vi "UHR-Fleezers Control (host) - 12.7e.vi"() -> ()   [LabVIEW 2012] (continued)
        n2981 = xnode "Read/Write Control"("FPGA VI Reference In"=w4045, "error in"=w4044) -> ("FPGA VI Reference Out"=w4043:T20, "error out"=w4042:errorcluster, "APD 3 Gate Late Counter"=→"APD 3 Gate Late Counter":u8, "APD 3 Gate Relative Phase"=→"APD 3 Gate Relative Phase":i16)
      }
    }
    n2982 = Not Equal?(x=w3728, y="Calibration") -> (x != y?=w3687:bool)
    n2983 = case shown="True" w3687 {
      tunnel: w3726 -> [_ w4076]
      tunnel: w3725 -> [_ w4075]
      tunnel: w3724 -> [_ w4074]
      tunnel: w3721 -> [_ w4073]
      tunnel: w3661 -> [_ w4072]
      frame False {
      }
      frame True {
        n2984 = property on="Force" class="WFChart (strict)"("YScale.NameLbl.Text"=w4076) -> ()  [unwired: 2 in, 2 out]
        n2985 = property on="T2 X" class="DigNum (strict)"("Caption.Text"=w4074) -> ()  [unwired: 2 in, 2 out]
        n2986 = property on="T1 X" class="DigNum (strict)"("Caption.Text"=w4075) -> ()  [unwired: 2 in, 2 out]
        n2987 = property on="Mean" class="DigNum (strict)"("Caption.Text"=w4073) -> ()  [unwired: 2 in, 2 out]
        n2988 = property on="Difference" class="DigNum (strict)"("Caption.Text"=w4072) -> ()  [unwired: 2 in, 2 out]
      }
    }
    n2989 = Unbundle By Name(w3709) -> ("Y"=w3712:dbl[])
    n2990 = Unbundle By Name(w3706) -> ("Y"=w3715:dbl[])
    n2991 = Subtract(x=w3712, y=w3710) -> (x-y=w3713:dbl[])
    n2992 = Subtract(x=w3715, y=w3708) -> (x-y=w3714:dbl[])
    n2993 = Multiply(x=w3714, y="T2 alpha_x (nm/V)") -> (x*y=w3510:dbl[])
    n2994 = Multiply(x="T1 alpha_x (nm/V)", y=w3713) -> (x*y=w3511:dbl[])
    n2995 = Not(x="Trap Trig. Fl.") -> (.not. x?=w3547:bool)
    n2996 = Multiply(x=w3736, y=-1.0) -> (x*y=w3717:waveform(dbl))
    n2997 = Subtract(x=w3511, y=w3510) -> (x-y=w3705:dbl[])
    n2998 = Unbundle By Name(w3736) -> ("Y"=w3677:dbl[])
    n2999 = Unbundle By Name(w3737) -> ("Y"=w3512:dbl[])
    n3000 = Negate(x=w3705) -> (-x=w3508:dbl[])
    n3001 = Build Array(w3737, w3717) -> (→"Force":waveform(dbl)[])
    n3002 = Subtract(x=w3508, y="Offset (nm)") -> (x-y=w3675:dbl[])
    n3003 = call-poly <vilib>:"Mean.vi"("X"=w3677) -> ("mean"=w3514:dbl)  [unwired: 1 out]
    "T2 X" <- w3514
    n3004 = Negate(x=w3677) -> (-x=w3678:dbl[])
    n3005 = call-poly <vilib>:"Mean.vi"("X"=w3512) -> ("mean"=w3515:dbl)  [unwired: 1 out]
    "T1 X" <- w3515
    n3006 = Negate(x=w3514) -> (-x=w3513:dbl)
    n3007 = Bundle By Name(cluster=w3709, "Y"=w3675) -> (w3653:waveform(dbl))
    "Bead Separation" <- w3653
    n3008 = Add(x=w3512, y=w3678) -> (x+y=w3679:dbl[])
    n3009 = Add(x=w3515, y=w3513) -> (x+y=w3723:dbl)
    n3010 = Subtract(x=w3515, y=w3513) -> (x-y=→"Difference":dbl)
    n3011 = Divide(x=w3679, y=2.0) -> (x/y=→"Vec Mean of T1 T2":dbl[])
    n3012 = Divide(x=w3723, y=2.0) -> (x/y=w3681:dbl)
    "Mean" <- w3681
    n3013 = feedback-in #25("Trap Trig. Fl.") -> ()
    n3014 = feedback #25("Trap Trig. Fl.") -> (w3545:bool)
    n3015 = And(x=w3547, y=w3545) -> (x .and. y?=w3546:bool)
    n3016 = case "If have just turned off triggering" shown="True" w3546 {
      tunnel: w3528 -> [_ w3873]
      tunnel: w3527 -> [_ w3872]
      frame False {
      }
      frame True {
        w3871 = FALSE ("FPGA Trap Trig")
        n3017 = xnode "Read/Write Control"("FPGA VI Reference In"=w3873, "error in"=w3872, "FPGA Trap Trig"=w3871) -> ("FPGA VI Reference Out"=w3870:T20, "error out"=w3869:errorcluster)
        n3018 = xnode "Read/Write Control"("FPGA VI Reference In"=w3870, "error in"=w3869, "TTrig?"=w3871) -> ()  [unwired: 2 out]
        n3019 = local write "Initializing"(FALSE ("Initializing")) -> ()
        n3020 = local write "Triggered"(FALSE ("Triggered")) -> ()
        n3021 = local write "Waiting"(FALSE ("Waiting")) -> ()
      }
    }
    n3022 = Not(x=w3545) -> (.not. x?=w3558:bool)
    n3023 = And(x="Trap Trig. Fl.", y=w3558) -> (x .and. y?=w3555:bool)
    n3024 = local read "Tether"() -> (w3682:bool)
    n3025 = Or(x=w3555, y="Reinitialize") -> (x .or. y?=w3541:bool)
    n3026 = feedback #26(w3551) -> (w3556:string)
    n3027 = Select(t=w3551, s=w3555, f=w3556) -> (s? t:f=w3550:string)
    n3028 = Select(t=w3551, s="Reinitialize", f=w3550) -> (s? t:f=w3549:string)
    n3029 = feedback #27(0) -> (w3553:i32)
    n3030 = feedback #28(w3675) -> (w3674:dbl[])
    n3031 = Build Array (concatenate)(w3675, w3674) -> (w3509:dbl[])
    n3032 = case "For determining if there is a tether still" shown="True" w3682 {
      tunnel: w3681 -> [_ w3997]
      frame False {
      }
      frame True {
        n3033 = Greater?(x="Lost Tether Alarm Threshold (pN)", y=w3997) -> (0:w3995:bool)
        n3034 = case shown="True" w3995 {
          frame False {
          }
          frame True {
            w3998 = FALSE ("Value (Signaling)")
            n3035 = flat-sequence {
              frame #0 {
                # "stop only if saving"
                n3036 = local read "Saving..."() -> (w4010:bool)
                n3037 = And(x=w4010, y="TA Cancel Save?") -> (x .and. y?=w4009:bool)
                n3038 = local write "Stop Saving"(w4009) -> ()
              }
              frame #1 {
                n3039 = case shown="True" "TA Green Off?" {
                  frame False {
                  }
                  frame True {
                    w4013 = FALSE ("Fl. Triggered...")
                    n3040 = local write "Fl. Triggered..."(w4013) -> ()
                    n3041 = property on="Green Laser ON" class="Bool (strict)"("Val(Sgnl)"=w4013) -> ()  [unwired: 2 in, 2 out]
                  }
                }
              }
            }
            n3042 = local read "Time tether formed"() -> (w4004:timestamp)
            n3043 = Get Date/Time In Seconds() -> (seconds since 1Jan1904=w4005:timestamp)
            n3044 = Subtract(x=w4005, y=w4004) -> (x-y=w4003:dbl)
            n3045 = Number To Decimal String(number=w4003) -> (decimal integer string=w4000:string)  [unwired: 1 out]
            n3046 = local read "Messages"() -> (w4007:string)
            n3047 = call <vilib>:"Beep.vi"() -> ()  [unwired: 3 in, 9 out]
            n3048 = Concatenate Strings("Lost tether (" ("Message to add"), w4000, " s)." ("string")) -> (w4002:string)
            n3049 = local write "Tether"(FALSE ("Tether")) -> ()
            n3050 = call "Update messages.vi"("Message to add"=w4002, "Old message string"=w4007) -> ("New message string"=w4006:string)
            n3051 = local write "Messages"(w4006) -> ()
            n3052 = property on="Fl. Triggered..." class="Bool (strict)"("Val(Sgnl)"=w3998) -> ()  [unwired: 2 in, 2 out]
            n3053 = local write "Dip for Protein"(w3998) -> ()
            n3054 = property on="Trap Pos. FB ON" class="Bool (strict)"("Val(Sgnl)"=w3998) -> ()  [unwired: 2 in, 2 out]
            n3055 = property on="Trap Trig. Fl." class="Bool (strict)"("Val(Sgnl)"=w3998) -> ()  [unwired: 2 in, 2 out]
          }
        }
      }
    }
    n3056 = case "For triggering actions based on the trap position (e.g., turning the excitation laser on if trap under feedback moves so far)" shown="True" "Trap Trig. Fl." {
      tunnel: w3536 -> [_ w3886]
      tunnel: w3549 -> [_ w3885]
      tunnel: ["" ("t") w3884] -> w3557
      tunnel: w3541 -> [_ w3883]
      tunnel: [0 ("t") w3882] -> w3554
      tunnel: w3553 -> [_ w3881]
      tunnel: w3528 -> [_ w3880]
      tunnel: w3527 -> [_ w3879]
      frame False {
      }
      frame True {
        n3057 = case shown="\"Wait for trigger\"" w3885 {
          tunnel: w3886 -> [w3903 _ _ w3951]
          tunnel: [w3900 w3932 "" ("t") w3954] -> w3884
          tunnel: w3883 -> [_ _ _ w3942]
          tunnel: [w3899 w3929 0 ("t") w3943] -> w3882
          tunnel: w3881 -> [_ w3931 _ w3949]
          tunnel: w3880 -> [w3888 w3926 _ w3945]
          tunnel: w3879 -> [w3887 w3925 _ w3944]
          frame "Wait for trigger" {
            n3058 = local read "Trap Trig. (FPGA)"() -> (w3891:bool)
            n3059 = Subtract(x=w3903, y="Mean T1 Position\nto compare (nm)") -> (x-y=w3896:dbl[])
            n3060 = call <vilib>:"Std Deviation and Variance.vi"("X"=w3896) -> ("mean"=→"mean":dbl, "standard deviation"=→"standard\ndeviation":dbl)  [unwired: 1 in, 1 out]
            n3061 = Array Max & Min(array=w3896) -> (max value=→"max value":dbl, min value=→"min value":dbl)  [unwired: 2 out]
            n3062 = Greater?(x=w3896, y="Threshold (nm)") -> (0:w3906:bool[])
            n3063 = case shown="True" w3891 {
              tunnel: w3888 -> [_ w3912]
              tunnel: w3887 -> [_ w3911]
              tunnel: [FALSE ("TTrig?") w3910] -> w3894
              frame False {
              }
              frame True {
                n3064 = xnode "Read/Write Control"("FPGA VI Reference In"=w3912, "error in"=w3911) -> ("TTrig?"=w3910:bool)  [unwired: 2 out]
              }
            }
            n3065 = Or Array Elements(Boolean array=w3906) -> (logical OR=w3893:bool)
            n3066 = Select(t=w3894, s=w3891, f=w3893) -> (s? t:f=w3892:bool)
            n3067 = Not(x=w3891) -> (.not. x?=w3890:bool)
            n3068 = And(x=w3892, y=w3890) -> (x .and. y?=w3889:bool)
            n3069 = Select(t="Triggered", s=w3892, f="Wait for trigger") -> (s? t:f=w3900:string)
            n3070 = case shown="True" w3892 {
              tunnel: [0 0] -> w3899
              tunnel: w3888 -> [_ w3917]
              tunnel: w3887 -> [_ w3916]
              frame False {
                "Waiting" <- TRUE ("Waiting")
              }
              frame True {
                n3071 = xnode "Read/Write Control"("FPGA VI Reference In"=w3917, "error in"=w3916, "TTrig?"=FALSE) -> ()  [unwired: 2 out]
                n3072 = local read "Messages"() -> (w3920:string)
                n3073 = call <vilib>:"Beep.vi"() -> ()  [unwired: 12 in]
                n3074 = call "Update messages.vi"("Message to add"="Unwinding trigger.", "Old message string"=w3920) -> ("New message string"=w3921:string)
                n3075 = local write "Messages"(w3921) -> ()
                n3076 = local write "Waiting"(FALSE ("Waiting")) -> ()
                "Triggered" <- TRUE ("Triggered")
              }
            }
            n3077 = case "Only need to turn on laser if host triggered" shown="True" w3889 {
              frame False {
              }
              frame True {
                n3078 = property on="Green Laser ON" class="Bool (strict)"("Val(Sgnl)"=TRUE ("Value (Signaling)")) -> ()  [unwired: 2 in, 2 out]
              }
            }
          }
          frame "Triggered" {
            n3079 = local read "Trap Trig. (FPGA)"() -> (w3928:bool)
            n3080 = Increment(x=w3931) -> (x+1=w3929:i32)
            n3081 = Greater Or Equal?(x=w3929, y="Fl. ON time (n)") -> (x >= y?=w3927:bool)
            n3082 = Select(t="Wait for trigger", s=w3927, f="Triggered" ("t")) -> (s? t:f=w3932:string)
            n3083 = And(x=w3927, y=w3928) -> (x .and. y?=w3924:bool)
            n3084 = case shown="True" w3924 {
              tunnel: w3926 -> [_ w3936]
              tunnel: w3925 -> [_ w3935]
              frame False {
              }
              frame True {
                n3085 = xnode "Read/Write Control"("FPGA VI Reference In"=w3936, "error in"=w3935, "FPGA Trap Trig"=TRUE) -> ()  [unwired: 2 out]
              }
            }
            n3086 = case shown="True" w3927 {
              frame False {
              }
              frame True {
                w3938 = FALSE ("Value (Signaling)")
                n3087 = local write "Triggered"(w3938) -> ()
                n3088 = local write "Waiting"(TRUE ("Waiting")) -> ()
                n3089 = property on="Green Laser ON" class="Bool (strict)"("Val(Sgnl)"=w3938) -> ()  [unwired: 2 in, 2 out]
              }
            }
          }
          frame "Do nothing" {
          }
          frame "Initialize", Default {
            n3090 = Increment(x=w3949) -> (x+1=w3953:i32)
            n3091 = Select(t=1, s=w3942, f=w3953) -> (s? t:f=w3943:i32)
            n3092 = feedback #29(w3951) -> (w3957:dbl[])
            n3093 = Build Array (concatenate)(w3951, w3957) -> (w3950:dbl[])
            n3094 = Greater Or Equal?(x=w3943, y="Wait to get offset (n)") -> (x >= y?=w3946:bool)
            n3095 = Select(t=w3951, s=w3942, f=w3950) -> (s? t:f=w3952:dbl[])
            n3096 = feedback-in #29(w3952) -> ()
            n3097 = call-poly <vilib>:"Mean.vi"("X"=w3952) -> ("mean"=w3947:dbl)  [unwired: 1 out]
            n3098 = local write "Mean T1 Position\nto compare (nm)"(w3947) -> ()
            n3099 = case shown="True" w3942 {
              tunnel: w3945 -> [_ w3963]
              tunnel: w3944 -> [_ w3962]
              frame False {
              }
              frame True {
                w3959 = FALSE ("FPGA Trap Trig")
                n3100 = xnode "Read/Write Control"("FPGA VI Reference In"=w3963, "error in"=w3962, "FPGA Trap Trig"=w3959) -> ("FPGA VI Reference Out"=w3961:T20, "error out"=w3960:errorcluster)
                n3101 = xnode "Read/Write Control"("FPGA VI Reference In"=w3961, "error in"=w3960, "TTrig?"=w3959) -> ()  [unwired: 2 out]
              }
            }
            n3102 = Select(t="Wait for trigger", s=w3946, f="Initialize") -> (s? t:f=w3954:string)
            n3103 = case shown="True" w3946 {
              tunnel: w3947 -> [_ w3966]
              tunnel: w3945 -> [_ w3975]
              tunnel: w3944 -> [_ w3974]
              frame False {
                n3104 = local write "Waiting"(FALSE ("Waiting")) -> ()
                "Initializing" <- TRUE ("Initializing")
              }
              frame True {
                n3105 = local read "Threshold (nm)"() -> (w3978:dbl)
                n3106 = local read "AOM X Cal (nm/MHz)"() -> (w3977:dbl)
                n3107 = Add(x=w3966, y=w3978) -> (x+y=w3979:dbl)
                n3108 = Divide(x=w3979, y=w3977) -> (x/y=w3976:dbl)
                n3109 = call "IR AOM freq to word.vi"("Frequency In (MHz)"=w3976) -> ("Frequency Word Out (double)"=w3973:dbl)
                n3110 = local write "Initializing"(FALSE ("Initializing")) -> ()
                n3111 = local write "Waiting"(TRUE ("Waiting")) -> ()
                n3112 = To Quad Integer(1:w3973) -> (0:w3972:i64)
                n3113 = xnode "Read/Write Control"("FPGA VI Reference In"=w3975, "error in"=w3974, "FPGA TTrig Thresh"=w3972) -> ("FPGA VI Reference Out"=w3969:T20, "error out"=w3968:errorcluster)
                n3114 = xnode "Read/Write Control"("FPGA VI Reference In"=w3969, "error in"=w3968, "FPGA Trap Trig"=TRUE) -> ()  [unwired: 2 out]
              }
            }
          }
        }
      }
    }
    n3115 = feedback-in #26(w3557) -> ()
    n3116 = feedback-in #27(w3554) -> ()
    n3117 = Split 1D Array(array=w3509, index=w3571) -> (first subarray=w3671:dbl[])  [unwired: 1 out]
    n3118 = feedback-in #28(w3671) -> ()
    n3119 = call-poly <vilib>:"Mean.vi"("X"=w3671) -> ("mean"=w3670:dbl)  [unwired: 1 out]
    "Bead Mean (nm)" <- w3670
    n3120 = Subtract(x=w3671, y=w3670) -> (x-y=w3669:dbl[])
    n3121 = Square(x=w3669) -> (x^2=w3668:dbl[])
    n3122 = call-poly <vilib>:"Mean.vi"("X"=w3668) -> ("mean"=w3667:dbl)  [unwired: 1 out]
    n3123 = Square Root(x=w3667) -> (sqrt(x)=w3666:dbl)
    n3124 = Multiply(x=10.0, y=w3666) -> (x*y=→"RMS (Ang)":dbl)
    n3125 = xnode ("Read/Write Control")("FPGA VI Reference In"=w3703, "error in"=w3702) -> ("FPGA VI Reference Out"=w3539:T20, "error out"=w3538:errorcluster, "AI2 Y Sum Set 1"=w3800:i16, "AI2 Y Sum Set 2"=w3799:i16, "AI1 X Set 1"=w3603:fxp<+/-,16,1>, "AI1 X Set 2"=w3602:fxp<+/-,16,1>, "Trap Pos FB Int Signal"=→"Trap Pos FB Int Signal":fxp<+/-,24,9>, "Trap Pos FB Int-Norm Signal"=→"Trap Pos FB Int-Norm Signal":fxp<+/-,16,1>, "Trap Pos FB Action"=w3596:i64, "Scanning"=→"AOD Scanning":bool, "Scan I"=→"AOD Scan I":u64, "Scanning MCL"=w3802:bool, "Scan I (MCL)"=→"MCL Scan I":u64, "Green FB Sum"=w3740:i16, "Trap Pos FB Action"=w3526:i64, "TTrig Fin Thresh"=w3522:i64, "Red FB Intensity"=w3503:i16, "Blue Intensity"=w3498:i16)
    "MCL Scanning" <- w3802
    "Trap Pos FB Action" <- w3596
    n3126 = Divide(x=w3503, y=3276.7) -> (x/y=w3502:dbl)
    "Red laser intensity (V)" <- w3502
    n3127 = Divide(x=w3498, y=3276.7) -> (x/y=w3497:dbl)
    "Blue laser intensity (V)" <- w3497
    n3128 = Divide(x=w3740, y=3276.7) -> (x/y=w3501:dbl)
    "Green laser intensity (V)" <- w3501
    n3129 = local read "FB Trig Integrate"() -> (w3520:u32)
    n3130 = Divide(x=w3526, y=w3520) -> (x/y=w3519:dbl)
    "TTrig Sig (Int)" <- w3519
    n3131 = Bundle(w3501, w3502, w3497) -> (→"Fluorescence laser intensities plot":cluster{dbl, dbl, dbl})  [unwired: 1 in]
    n3132 = Divide(x=w3522, y=w3520) -> (x/y=w3517:dbl)
    "TTrig Fin Thresh (Int)" <- w3517
    n3133 = local read "AOM X Cal (nm/MHz)"() -> (w3525:dbl)
    n3134 = local read "AI2 (V)"() -> (w3801:cluster{"Set 1":dbl, "Set 2":dbl})
    n3135 = Bundle By Name(cluster=w3801, "Set 1"=w3800, "Set 2"=w3799) -> (w3797:cluster{"Set 1":dbl, "Set 2":dbl})
    n3136 = Divide(x=w3596, y=327.67) -> (x/y=→"Action (%)":dbl)
    n3137 = local read "Trap X (AI1)"() -> (w3616:T10)
    n3138 = call "IR AOM word double to freq.vi"("Frequency Word In (double)"=w3517) -> ("Frequency Out (MHz)"=w3516:dbl)
    n3139 = call "IR AOM word double to freq.vi"("Frequency Word In (double)"=w3519) -> ("Frequency Out (MHz)"=w3518:dbl)
    n3140 = Divide(x=w3797, y=3276.7) -> (x/y=w3796:cluster{"Set 1":dbl, "Set 2":dbl})
    n3141 = Multiply(x=w3518, y=w3525) -> (x*y=w3524:dbl)
    "TTrig Sig (nm)" <- w3524
    n3142 = Multiply(x=w3516, y=w3525) -> (x*y=w3523:dbl)
    "TTrig Fin Thresh (nm)" <- w3523
    n3143 = local write "AI2 (V)"(w3796) -> ()
    n3144 = Bundle(cluster=w3616, "Trap 1"=w3603, "Trap 2"=w3602) -> (→"Trap X (AI1)":T10)
    n3145 = Bundle(w3524, w3523) -> (→"TTrig":cluster{dbl, dbl})  [unwired: 1 in]
    n3146 = flat-sequence "To save data" {
      tunnel: [w4886] -> w3820
      tunnel: [w4887] -> w3819
      tunnel: w3771 -> [w4880]
      tunnel: w3544 -> [w4884]
      tunnel: ["Save Calibration"] -> w3793
      tunnel: w3790 -> [w4883]
      tunnel: [w4876] -> w3789
      tunnel: [w4873] -> w3788
      tunnel: [w4870] -> w3787
      tunnel: w3770 -> [w4872]
      tunnel: w3685 -> [w4866]
      tunnel: [w4866] -> w3684
      tunnel: ["Start Saving"] -> w3654
      tunnel: [w4860] -> w3584
      tunnel: [w4859] -> w3583
      tunnel: w3820 -> [w5134]
      tunnel: w3819 -> [w5133]
      tunnel: w3585 -> [w5132]
      tunnel: w3793 -> [w5131]
      tunnel: w3789 -> [w5129]
      tunnel: w3788 -> [w5128]
      tunnel: w3787 -> [w5127]
      tunnel: w3663 -> [w5126]
      tunnel: w3695 -> [w5125]
      tunnel: w3684 -> [w5124]
      tunnel: w3654 -> [w5123]
      tunnel: w3653 -> [w5122]
      tunnel: w3483 -> [w5121]
      tunnel: w3584 -> [w5120]
      tunnel: w3583 -> [w5119]
      tunnel: w3582 -> [w5118]
      tunnel: w3505 -> [w5117]
      frame #0 {
        n3147 = Or(x="Save N Sets", y="Start Saving") -> (x .or. y?=w4867:bool)
        n3148 = To Double Precision Float(number=w4883) -> (double precision float=w4877:dbl)
        n3149 = Build Array(w4867, "Save Calibration", w4880, w4872) -> (w4882:bool[])
        n3150 = Compound Arithmetic op=OR("Save Calibration", w4880, w4867, w4872) -> (w4885:bool)
        n3151 = Boolean Array To Number(Boolean array=w4882) -> (number=w4879:u32)
        n3152 = feedback #30(FALSE ("Save APD Data\nwith Trap Data")) -> (w4861:bool)
        n3153 = feedback #31(refnum<k0> refnum) -> (w4888:refnum<file>)
        n3154 = feedback #32(refnum<k0> refnum) -> (w4863:refnum<file>)
        n3155 = feedback #33(FALSE ("Save APD Data\nwith Trap Data")) -> (w4871:bool)
        n3156 = feedback #34(refnum<k0> refnum) -> (w4874:refnum<file>)
        n3157 = feedback #35(0) -> (w4890:i32)
        n3158 = feedback #36() -> (w4878:u32)  [unwired: 1 out]
        n3159 = case shown="True" w4885 {
          tunnel: [w4897 1] -> w4886
          tunnel: w4890 -> [w4899 _]
          tunnel: [w4898 w4930] -> w4887
          tunnel: w4888 -> [w4898 _]
          tunnel: w4884 -> [_ w4948]
          tunnel: w4877 -> [_ w4946]
          tunnel: w4879 -> [_ w4949]
          tunnel: [w4896 w4929] -> w4876
          tunnel: w4878 -> [w4896 _]
          tunnel: [w4895 w4927] -> w4873
          tunnel: w4874 -> [w4895 _]
          tunnel: [w4894 w4926] -> w4870
          tunnel: w4871 -> [w4894 _]
          tunnel: "Start Saving" -> [_ w4924]
          tunnel: w4866 -> [_ w4923]
          tunnel: [w4893 w4915] -> w4859
          tunnel: w4863 -> [w4893 _]
          tunnel: [w4892 w4914] -> w4860
          tunnel: w4861 -> [w4892 _]
          frame False {
            n3160 = Increment(x=w4899) -> (x+1=w4897:i32)
          }
          frame True {
            w4920 = FALSE ("Start Saving")
            w4925 = 9.0  # File Version
            w4932 = FALSE ("prepend array or string size? (T)")
            w4931 = T26."big-endian, network order" ("byte order (0:big-endian, network order)")
            n3161 = local read "BD 1 Frequency 1 (MHz)"() -> (w4945:dbl)
            n3162 = local read "BD 2 Frequency 1 (MHz)"() -> (w4944:dbl)
            n3163 = local read "BD 1 Frequency 2 (MHz)"() -> (w4943:dbl)
            n3164 = local read "BD 2 Frequency 2 (MHz)"() -> (w4942:dbl)
            n3165 = local read "BD 1 Frequency 3 (MHz)"() -> (w4941:dbl)
            n3166 = local read "BD 2 Frequency 3 (MHz)"() -> (w4940:dbl)
            n3167 = Array Size(array=w4923) -> (size(s)=w4922:i32)
            n3168 = To Double Precision Float(number=w4922) -> (double precision float=w4921:dbl)
            n3169 = local write "Save Calibration"(w4920) -> ()
            n3170 = local write "Start Saving"(w4920) -> ()
            n3171 = Build Array("Save APD Data\nwith Trap Data", "Save Trap Pos. Data") -> (w4917:bool[])
            n3172 = Boolean Array To Number(Boolean array=w4917) -> (number=w4916:u32)
            n3173 = Build Array(w4945, w4944, w4943, w4942, w4941, w4940) -> (w4939:dbl[])
            n3174 = case shown="1, Default" w4949 {
              tunnel: w4948 -> [w5021 w5041 w5057 w5095]
              tunnel: w4921 -> [w5026 w5048 w5077 w5114]
              tunnel: w4946 -> [w5025 w5047 w5076 w5113]
              tunnel: [w5022 w5043 w5068 w5105] -> w4937
              tunnel: [w5013 "Cal sets to save" w5058 w5096] -> w4929
              tunnel: w4939 -> [w5023 w5044 w5070 w5107]
              tunnel: "Save APD Data\nwith Trap Data" -> [w5020 _ w5054 w5093]
              tunnel: [w5020 w5035 w5054 w5093] -> w4926
              tunnel: w4925 -> [w5016 w5036 w5052 w5091]
              tunnel: w4924 -> [w5015 _ _ _]
              tunnel: [w5006 w5035 w5051 w5081] -> w4914
              tunnel: "Save Trap Pos. Data" -> [w5006 _ w5051 w5081]
              tunnel: w4916 -> [w5005 _ w5050 w5080]
              frame 1, Default {
                # "timeseries"
                n3175 = case shown="True" "Profile" {
                  tunnel: [w5029 w5033] -> w5010
                  tunnel: [w5029 w5032] -> w5009
                  tunnel: [w5029 w5031] -> w5008
                  tunnel: [w5029 w5030] -> w5007
                  frame False {
                    w5029 = 0.0 ("f")
                  }
                  frame True {
                    n3176 = local read "Current Position"() -> (w5034:cluster{dbl, dbl, dbl})
                    n3177 = local read "Y change (mm)"() -> (w5030:dbl)
                    n3178 = Unbundle(w5034) -> (w5033:dbl, w5032:dbl, w5031:dbl)
                  }
                }
                n3179 = local read "Save ave N"() -> (w5028:dbl)
                n3180 = Multiply(x=w5028, y=w5021) -> (x*y=w5027:dbl)
                n3181 = To Double Precision Float(number=w5005) -> (double precision float=w5019:dbl)
                n3182 = Build Array(w5016, w5021, w5027, w5026, w5025, 0.0 ("f")) -> (w5024:dbl[])
                n3183 = Build Array(w5019, w5010, w5009, w5008, w5007) -> (w5017:dbl[])
                n3184 = Select(t=u32 4000000000, s=w5015, f="N sets to save") -> (s? t:f=w5013:u32)
                n3185 = Build Array (concatenate)(w5024, w5023, w5017) -> (w5022:dbl[])
              }
              frame 2 {
                w5038 = 0.0 ("f")
                w5035 = FALSE ("Save APD Data\nwith Trap Data")
                # "calibration"
                n3186 = Boolean To (0,1)(Boolean=w5035) -> (0, 1=w5040:i16)
                n3187 = To Double Precision Float(number=w5040) -> (double precision float=w5039:dbl)
                n3188 = Build Array(w5039, w5038, w5038, w5038, w5038) -> (w5037:dbl[])
                n3189 = Build Array(w5036, w5041, w5041, w5048, w5047, 1.0 ("t")) -> (w5045:dbl[])
                n3190 = Build Array (concatenate)(w5045, w5044, w5037) -> (w5043:dbl[])
                "Calibrating Trap..." <- TRUE ("Calibrating...")
              }
              frame 4 {
                w5055 = 0.0 ("f")
                # "scan dir (x/y = 0/1)"
                # "cycles/step"
                # "n scans (f/b)"
                # "steps"
                # "freq. range"
                # "AOD raster scan"
                n3191 = local read "Number of F/B Scans (AOD)"() -> (w5062:u16)
                n3192 = local read "Cycles/step (AOD)"() -> (w5064:u64)
                n3193 = local read "Scan Range (MHz)"() -> (w5067:dbl)
                n3194 = local read "Scan steps (AOD)"() -> (w5066:u64)
                n3195 = local read "Scan BD"() -> (w5074:bool)
                n3196 = local read "Save ave N"() -> (w5079:dbl)
                n3197 = Boolean To (0,1)(Boolean=w5074) -> (0, 1=w5073:i16)
                n3198 = To Double Precision Float(number=w5062) -> (double precision float=w5061:dbl)
                n3199 = To Double Precision Float(number=w5066) -> (double precision float=w5065:dbl)
                n3200 = To Double Precision Float(number=w5064) -> (double precision float=w5063:dbl)
                n3201 = To Double Precision Float(number=w5073) -> (double precision float=w5072:dbl)
                n3202 = Multiply(x=w5079, y=w5057) -> (x*y=w5078:dbl)
                n3203 = To Double Precision Float(number=w5050) -> (double precision float=w5056:dbl)
                n3204 = Build Array(w5056, w5055, w5055, w5055, w5055) -> (w5053:dbl[])
                n3205 = local read "N sets should be saved"() -> (w5059:dbl)
                n3206 = Build Array(w5072, w5067, w5065, w5063, w5061) -> (w5069:dbl[])
                n3207 = Build Array(w5052, w5057, w5078, w5077, w5076, 2.0 ("t")) -> (w5071:dbl[])
                n3208 = Round Toward +Infinity(x=w5059) -> (ceil(x): smallest int >= x=w5060:dbl)
                n3209 = Build Array (concatenate)(w5071, w5070, w5053, w5069) -> (w5068:dbl[])
                n3210 = To Unsigned Long Integer(number=w5060) -> (unsigned 32bit integer=w5058:u32)
              }
              frame 8 {
                w5088 = 0.0 ("f")
                # "MCL raster scan"
                n3211 = local read "Number of scans (MCL)"() -> (w5083:u64)
                n3212 = local read "Scan lines (y)"() -> (w5082:u64)
                n3213 = local read "2D or 1D Scan"() -> (w5085:bool)
                n3214 = local read "Scan Range (V)\n(of steps)"() -> (w5104:dbl)
                n3215 = local read "Fast Scan Dir"() -> (w5111:bool)
                n3216 = local read "Cycles/step (MCL)"() -> (w5101:u64)
                n3217 = local read "Scan steps (MCL)"() -> (w5103:u64)
                n3218 = Select(t=w5082, s=w5085, f=w5083) -> (s? t:f=w5084:u64)
                n3219 = Boolean To (0,1)(Boolean=w5085) -> (0, 1=w5087:i16)
                n3220 = local read "Save ave N"() -> (w5116:dbl)
                n3221 = local read "Initial X"() -> (w5090:dbl)
                n3222 = local read "Initial Y"() -> (w5089:dbl)
                n3223 = To Double Precision Float(number=w5087) -> (double precision float=w5086:dbl)
                n3224 = Boolean To (0,1)(Boolean=w5111) -> (0, 1=w5110:i16)
                n3225 = To Double Precision Float(number=w5084) -> (double precision float=w5099:dbl)
                n3226 = To Double Precision Float(number=w5103) -> (double precision float=w5102:dbl)
                n3227 = To Double Precision Float(number=w5101) -> (double precision float=w5100:dbl)
                n3228 = To Double Precision Float(number=w5110) -> (double precision float=w5109:dbl)
                n3229 = Multiply(x=w5116, y=w5095) -> (x*y=w5115:dbl)
                n3230 = To Double Precision Float(number=w5080) -> (double precision float=w5094:dbl)
                n3231 = local read "N sets should be saved (MCL)"() -> (w5097:dbl)
                n3232 = Build Array(w5094, w5086, w5088, w5088, w5088) -> (w5092:dbl[])
                n3233 = Build Array(w5109, w5104, w5102, w5100, w5099, w5090, w5089) -> (w5106:dbl[])
                n3234 = Build Array(w5091, w5095, w5115, w5114, w5113, 3.0 ("t")) -> (w5108:dbl[])
                n3235 = Round Toward +Infinity(x=w5097) -> (ceil(x): smallest int >= x=w5098:dbl)
                n3236 = Build Array (concatenate)(w5108, w5107, w5092, w5106) -> (w5105:dbl[])
                n3237 = To Unsigned Long Integer(number=w5098) -> (unsigned 32bit integer=w5096:u32)
              }
            }
            n3238 = local read "Index"() -> (w4954:dbl)
            n3239 = call "Create new save file.vi"("Insert"="", "Ext"=".dat", "Index In"=w4954) -> ("Path Out"=w4910:path, "Index Out"=w4928:dbl)
            n3240 = local write "Save file name"(w4910) -> ()
            n3241 = local write "Index"(w4928) -> ()
            n3242 = local write "Save index"(w4928) -> ()
            n3243 = Array Size(array=w4937) -> (size(s)=w4938:i32)
            n3244 = Open/Create/Replace File(file path (use dialog)=w4910, operation (0:open)=T27."create", access (0:read/write)=enum16{"read/write", "read-only", "write-only"}."write-only") -> (refnum out=w4951:refnum<file>)  [unwired: 1 in, 4 out]
            n3245 = local write "Saving..."(TRUE ("Saving...")) -> ()
            n3246 = To Double Precision Float(number=w4938) -> (double precision float=w4936:dbl)
            n3247 = String Length(string="Comment (data description)") -> (length=w4935:i32)
            n3248 = To Double Precision Float(number=w4935) -> (double precision float=w4934:dbl)
            n3249 = Deny Access(7:w4951) -> (3:w4950:refnum<file>)  [unwired: 1 in, 2 out]
            n3250 = Build Array (concatenate)(w4936, w4937, w4934) -> (w4909:dbl[])
            n3251 = case "If fluorescence data to be saved" shown="True" w4926 {
              tunnel: w4910 -> [_ w5004]
              tunnel: [refnum<k0> refnum w4984] -> w4927
              frame False {
              }
              frame True {
                w4983 = 0.0
                n3252 = local read "APD Integration Time (s)"() -> (w4989:dbl)
                n3253 = local read "N APD Samp/step"() -> (w4982:dbl)
                n3254 = local read "Number of APDs"() -> (w4981:u8)
                n3255 = Path To String(path=w5004) -> (string=w5003:string)
                n3256 = String Length(string=w5003) -> (length=w5002:i32)
                n3257 = Subtract(x=w5002, y=4) -> (x-y=w5000:i32)
                n3258 = String Subset(string=w5003, length (rest)=w5000) -> (substring=w4999:string)  [unwired: 1 out]
                n3259 = Build Array(w4989, w4982, w4981, w4983, w4983, w4983, w4983, w4983) -> (w4986:dbl[])
                n3260 = Concatenate Strings(w4999, "_fl.dat" ("string")) -> (w4997:string)
                n3261 = Array Size(array=w4986) -> (size(s)=w4988:i32)
                n3262 = String To Path(string=w4997) -> (path=w4993:path)
                n3263 = Open/Create/Replace File(file path (use dialog)=w4993, operation (0:open)=T27."create", access (0:read/write)=enum16{"read/write", "read-only", "write-only"}."write-only") -> (refnum out=w4994:refnum<file>)  [unwired: 1 in, 4 out]
                n3264 = Deny Access(7:w4994) -> (3:w4990:refnum<file>)  [unwired: 1 in, 2 out]
                n3265 = To Double Precision Float(number=w4988) -> (double precision float=w4987:dbl)
                n3266 = Build Array (concatenate)(w4987, w4986) -> (w4985:dbl[])
                n3267 = Write to Binary File(file (use dialog)=w4990, data=w4985, 5:FALSE ("prepend array or string size? (T)"), 9:T26."big-endian, network order" ("byte order (0:big-endian, network order)")) -> (refnum out=w4984:refnum<file>)  [unwired: 1 in, 3 out]
              }
            }
            n3268 = case shown="True" w4914 {
              tunnel: w4910 -> [_ w4965]
              tunnel: [refnum<k0> refnum w4964] -> w4915
              frame False {
              }
              frame True {
                w4960 = 0.0 ("element")
                n3269 = Path To String(path=w4965) -> (string=w4979:string)
                n3270 = Build Array(w4960, w4960, w4960, w4960, w4960, w4960, w4960, w4960) -> (w4961:dbl[])
                n3271 = String Length(string=w4979) -> (length=w4978:i32)
                n3272 = Subtract(x=w4978, y=4) -> (x-y=w4976:i32)
                n3273 = Array Size(array=w4961) -> (size(s)=w4963:i32)
                n3274 = String Subset(string=w4979, length (rest)=w4976) -> (substring=w4975:string)  [unwired: 1 out]
                n3275 = To Double Precision Float(number=w4963) -> (double precision float=w4962:dbl)
                n3276 = Concatenate Strings(w4975, "_pos.dat" ("string")) -> (w4973:string)
                n3277 = Build Array (concatenate)(w4962, w4961) -> (w4959:dbl[])
                n3278 = String To Path(string=w4973) -> (path=w4969:path)
                n3279 = Open/Create/Replace File(file path (use dialog)=w4969, operation (0:open)=T27."create", access (0:read/write)=enum16{"read/write", "read-only", "write-only"}."write-only") -> (refnum out=w4970:refnum<file>)  [unwired: 1 in, 4 out]
                n3280 = Deny Access(7:w4970) -> (3:w4966:refnum<file>)  [unwired: 1 in, 2 out]
                n3281 = Write to Binary File(file (use dialog)=w4966, data=w4959, 5:FALSE ("prepend array or string size? (T)"), 9:T26."big-endian, network order" ("byte order (0:big-endian, network order)")) -> (refnum out=w4964:refnum<file>)  [unwired: 1 in, 3 out]
              }
            }
            n3282 = Write to Binary File(file (use dialog)=w4950, data=w4909, 5:w4932, 9:w4931) -> (refnum out=w4933:refnum<file>)  [unwired: 1 in, 3 out]
            n3283 = Write to Binary File(file (use dialog)=w4933, data="Comment (data description)", 5:w4932, 9:w4931) -> (refnum out=w4930:refnum<file>)  [unwired: 1 in, 3 out]
            n3284 = local read "connection reference"() -> (w4912:T17)
            n3285 = Bundle("Comment (data description)"="Comment (data description)", "Channel 1 Buffer"="Channel 1 Buffer", "Channel 2 Buffer"="Channel 2 Buffer", "Channel 3 Buffer"="Channel 3 Buffer", "Title"="Title", "DNA Construct"="DNA Construct", "Bead diameter"="Bead diameter", "Name"="Name") -> (w4900:T50)  [unwired: 1 in]
            n3286 = call "MattFileCreator-v9.vi"("Comments"=w4900, "Input Array"=w4909, "File path"=w4910, "table"="labview", "connection reference"=w4912) -> ("connection reference out"=w4911:T17)  [unwired: 5 in, 1 out]
            n3287 = local write "connection reference"(w4911) -> ()
          }
        }
        n3288 = feedback-in #30(w4860) -> ()
        n3289 = feedback-in #31(w4887) -> ()
        n3290 = feedback-in #32(w4859) -> ()
        n3291 = feedback-in #33(w4870) -> ()
        n3292 = feedback-in #34(w4873) -> ()
        n3293 = feedback-in #35(w4886) -> ()
        n3294 = feedback-in #36(w4876) -> ()
      }
      frame #1 {
        n3295 = local read "Saving..."() -> (w5130:bool)
        n3296 = case shown="True" w5130 {
          tunnel: w5134 -> [_ w5145]
          tunnel: w5133 -> [_ w5159]
          tunnel: w5132 -> [_ w5155]
          tunnel: w5131 -> [_ w5154]
          tunnel: w5129 -> [_ w5153]
          tunnel: w5128 -> [_ w5148]
          tunnel: w5127 -> [_ w5147]
          tunnel: w5126 -> [_ w5146]
          tunnel: w5125 -> [_ w5144]
          tunnel: w5124 -> [_ w5142]
          tunnel: w5123 -> [_ w5141]
          tunnel: w5122 -> [_ w5140]
          tunnel: w5121 -> [_ w5139]
          tunnel: w5120 -> [_ w5138]
          tunnel: w5119 -> [_ w5137]
          tunnel: w5118 -> [_ w5136]
          tunnel: w5117 -> [_ w5135]
          frame False {
          }
          frame True {
            n3297 = Multiply(x=w5145, y=w5144) -> (x*y=→"Time (s)":dbl)
            n3298 = Less Or Equal?(x=w5145, y=w5153) -> (x <= y?=w5157:bool)
            n3299 = Or(x="Stop Saving", y="Abort save 2") -> (x .or. y?=w5149:bool)
            n3300 = Not(x=w5149) -> (.not. x?=w5158:bool)
            n3301 = And(x=w5157, y=w5158) -> (x .and. y?=w5156:bool)
            n3302 = case shown="True" w5156 {
              tunnel: w5159 -> [w5166 w5257]
              tunnel: [0.0 w5260] -> w5152
              tunnel: w5145 -> [_ w5258]
              tunnel: w5153 -> [_ w5259]
              tunnel: w5155 -> [_ w5254]
              tunnel: w5154 -> [_ _]
              tunnel: w5148 -> [w5164 w5247]
              tunnel: w5147 -> [w5163 w5248]
              tunnel: w5146 -> [_ w5246]
              tunnel: w5142 -> [_ w5245]
              tunnel: w5141 -> [_ w5169]
              tunnel: w5140 -> [_ w5238]
              tunnel: w5139 -> [_ w5185]
              tunnel: w5138 -> [w5160 w5202]
              tunnel: w5137 -> [w5161 w5201]
              tunnel: w5136 -> [_ w5198]
              tunnel: w5135 -> [_ w5196]
              frame False {
                w5162 = FALSE
                n3303 = Close File(refnum=w5166) -> ()  [unwired: 1 in, 2 out]
                n3304 = case shown="True" w5163 {
                  tunnel: w5164 -> [_ w5168]
                  frame False {
                  }
                  frame True {
                    n3305 = Close File(refnum=w5168) -> ()  [unwired: 1 in, 2 out]
                  }
                }
                n3306 = case shown="True" w5160 {
                  tunnel: w5161 -> [_ w5167]
                  frame False {
                  }
                  frame True {
                    n3307 = Close File(refnum=w5167) -> ()  [unwired: 1 in, 2 out]
                  }
                }
                n3308 = local write "Raster Scanning..."(w5162) -> ()
                n3309 = local write "Calibrating Trap..."(w5162) -> ()
                n3310 = call <vilib>:"Beep.vi"() -> ()  [unwired: 3 in, 9 out]
                n3311 = local write "Stop Saving"(w5162) -> ()
                "Saving..." <- w5162
              }
              frame True {
                n3312 = local read "Calibrating Trap..."() -> (w5249:bool)
                n3313 = case "Write fl. data" shown="True" w5248 {
                  tunnel: w5247 -> [_ w5283]
                  tunnel: w5246 -> [_ w5282]
                  frame False {
                  }
                  frame True {
                    n3314 = Write to Binary File(file (use dialog)=w5283, data=w5282, 5:FALSE ("prepend array or string size? (T)"), 9:T26."big-endian, network order" ("byte order (0:big-endian, network order)")) -> ()  [unwired: 1 in, 4 out]
                  }
                }
                n3315 = Greater?(x="Save ave N", y=1.0) -> (0:w5252:bool)
                n3316 = Not(x=w5249) -> (.not. x?=w5251:bool)
                n3317 = And(x=w5251, y=w5252) -> (x .and. y?=w5199:bool)
                n3318 = case shown="True" w5199 {
                  tunnel: w5198 -> [w5263 w5274]
                  tunnel: [w5263 w5266] -> w5197
                  tunnel: "Save ave N" -> [_ w5267]
                  frame False {
                  }
                  frame True {
                    w5264 = 2 ("dimension size")
                    n3319 = Array Size(array=w5274) -> (size(s)=w5268:i32)
                    n3320 = Divide(x=w5268, y=w5264) -> (x/y=w5272:dbl)
                    n3321 = Reshape Array(w5274, w5272, w5264) -> (w5273:u64[][])
                    n3322 = Transpose 2D Array(2D array=w5273) -> (transposed array=w5271:u64[][])
                    n3323 = for {
                      tunnel: w5271 -> [w5276] mode=indexing
                      tunnel: [w5275] -> w5265 mode=indexing
                      tunnel: w5267 -> [w5277]
                      workers-P: _ -> [_]
                      n3324 = call "downsample 1D array - U64.vi"("Ave N"=w5277, "Array In"=w5276) -> ("Array Out"=w5275:u64[])  [unwired: 1 in]
                    }
                    n3325 = Transpose 2D Array(2D array=w5265) -> (transposed array=w5270:u64[][])
                    n3326 = Divide(x=w5268, y=w5267) -> (x/y=w5269:dbl)
                    n3327 = Reshape Array(w5270, w5269) -> (w5266:u64[])
                  }
                }
                n3328 = case shown="True" w5199 {
                  tunnel: w5254 -> [w5286 w5298]
                  tunnel: [w5286 w5290] -> w5250
                  tunnel: "Save ave N" -> [_ w5291]
                  tunnel: w5245 -> [_ w5289]
                  frame False {
                  }
                  frame True {
                    n3329 = Array Size(array=w5298) -> (size(s)=w5292:i32)
                    n3330 = Array Size(array=w5289) -> (size(s)=w5288:i32)
                    n3331 = Divide(x=w5292, y=w5288) -> (x/y=w5296:dbl)
                    n3332 = Reshape Array(w5298, w5296, w5288) -> (w5297:i16[][])
                    n3333 = Transpose 2D Array(2D array=w5297) -> (transposed array=w5295:i16[][])
                    n3334 = for {
                      tunnel: w5295 -> [w5301] mode=indexing
                      tunnel: [w5300] -> w5287 mode=indexing
                      tunnel: w5291 -> [w5299]
                      workers-P: _ -> [_]
                      n3335 = call "downsample 1D array - I16.vi"("Ave N"=w5299, "Array In"=w5301) -> ("Array Out"=w5300:i16[])  [unwired: 1 out]
                    }
                    n3336 = Transpose 2D Array(2D array=w5287) -> (transposed array=w5294:i16[][])
                    n3337 = Divide(x=w5292, y=w5291) -> (x/y=w5293:dbl)
                    n3338 = Reshape Array(w5294, w5293) -> (w5290:i16[])
                  }
                }
                n3339 = Index Array(array=w5185, index=2) -> (element=w5186:waveform(dbl))
                n3340 = Index Array(array=w5185, index=1) -> (element=w5219:waveform(dbl))
                n3341 = Index Array(array=w5185, index=0) -> (element=w5221:waveform(dbl))
                n3342 = Unbundle By Name(w5186) -> ("Y"=w5188:dbl[])
                n3343 = Unbundle By Name(w5219) -> ("Y"=w5223:dbl[])
                n3344 = Unbundle By Name(w5221) -> ("Y"=w5231:dbl[])
                n3345 = case "Write trap pos. data" shown="True" w5202 {
                  tunnel: w5201 -> [_ w5279]
                  tunnel: w5197 -> [_ w5278]
                  frame False {
                  }
                  frame True {
                    n3346 = Write to Binary File(file (use dialog)=w5279, data=w5278, 5:FALSE ("prepend array or string size? (T)"), 9:T26."big-endian, network order" ("byte order (0:big-endian, network order)")) -> ()  [unwired: 1 in, 4 out]
                  }
                }
                n3347 = Write to Binary File(file (use dialog)=w5257, data=w5250, 5:FALSE ("prepend array or string size? (T)"), 9:T26."big-endian, network order" ("byte order (0:big-endian, network order)")) -> ()  [unwired: 1 in, 4 out]
                n3348 = feedback #37(w5188) -> (w5189:dbl[])
                n3349 = Build Array (concatenate)(w5189, w5188) -> (w5184:dbl[])
                n3350 = Select(t=w5188, s=w5169, f=w5184) -> (s? t:f=w5174:dbl[])
                n3351 = feedback-in #37(w5174) -> ()
                n3352 = feedback #38(w5223) -> (w5225:dbl[])
                n3353 = Build Array (concatenate)(w5225, w5223) -> (w5224:dbl[])
                n3354 = Select(t=w5223, s=w5169, f=w5224) -> (s? t:f=w5213:dbl[])
                n3355 = feedback-in #38(w5213) -> ()
                n3356 = feedback #39(w5231) -> (w5244:dbl[])
                n3357 = Build Array (concatenate)(w5244, w5231) -> (w5243:dbl[])
                n3358 = Select(t=w5231, s=w5169, f=w5243) -> (s? t:f=w5218:dbl[])
                n3359 = feedback-in #39(w5218) -> ()
                n3360 = Divide(x=w5258, y=w5259) -> (x/y=w5261:dbl)
                n3361 = Multiply(x=w5261, y=100.0) -> (x*y=w5260:dbl)
                n3362 = Build Array(w5218, w5213, w5174) -> (→"Saved APD":dbl[][])
                n3363 = Array Size(array=w5218) -> (size(s)=w5236:i32)
                n3364 = Unbundle By Name(w5238) -> ("Y"=w5242:dbl[])
                n3365 = Subtract(x=w5236, y="N pts to average") -> (x-y=w5171:i32)
                n3366 = Multiply(x="N pts to average", y=u16 2) -> (x*y=w5214:u16)
                n3367 = Subtract(x=w5236, y=w5214) -> (x-y=w5172:i32)
                n3368 = feedback #40(w5242) -> (w5241:dbl[])
                n3369 = Build Array (concatenate)(w5241, w5242) -> (w5240:dbl[])
                n3370 = Select(t=w5242, s=w5169, f=w5240) -> (s? t:f=w5239:dbl[])
                "Trap Delta Graph" <- w5239
                n3371 = feedback-in #40(w5239) -> ()
                n3372 = Array Subset(array=w5218, index=w5171, length="N pts to average") -> (w5235:dbl[])
                n3373 = Array Subset(array=w5218, index=w5172, length="N pts to average") -> (w5234:dbl[])
                n3374 = Array Subset(array=w5213, index=w5171, length="N pts to average") -> (w5216:dbl[])
                n3375 = Array Subset(array=w5213, index=w5172, length="N pts to average") -> (w5215:dbl[])
                n3376 = Array Subset(array=w5174, index=w5171, length="N pts to average") -> (w5183:dbl[])
                n3377 = Array Subset(array=w5174, index=w5172, length="N pts to average") -> (w5182:dbl[])
                n3378 = Index Array(array=w5196, index=0) -> (element=w5194:waveform(dbl))
                n3379 = call-poly <vilib>:"Mean.vi"("X"=w5235) -> ("mean"=w5233:dbl)  [unwired: 1 out]
                n3380 = call-poly <vilib>:"Mean.vi"("X"=w5216) -> ("mean"=w5212:dbl)  [unwired: 1 out]
                n3381 = call-poly <vilib>:"Mean.vi"("X"=w5234) -> ("mean"=w5232:dbl)  [unwired: 1 out]
                n3382 = call-poly <vilib>:"Mean.vi"("X"=w5215) -> ("mean"=w5211:dbl)  [unwired: 1 out]
                n3383 = call-poly <vilib>:"Mean.vi"("X"=w5183) -> ("mean"=w5181:dbl)  [unwired: 1 out]
                n3384 = call-poly <vilib>:"Mean.vi"("X"=w5182) -> ("mean"=w5180:dbl)  [unwired: 1 out]
                n3385 = Unbundle By Name(w5194) -> ("Y"=w5192:dbl[])
                n3386 = Subtract(x=w5212, y=w5211) -> (x-y=w5203:dbl)
                "Delta Fl. 2" <- w5203
                n3387 = Subtract(x=w5181, y=w5180) -> (x-y=w5175:dbl)
                "Delta Fl. 3" <- w5175
                n3388 = Subtract(x=w5233, y=w5232) -> (x-y=w5230:dbl)
                "Delta Fl. 1" <- w5230
                n3389 = feedback #41(w5192) -> (w5191:dbl[])
                n3390 = Build Array (concatenate)(w5191, w5192) -> (w5193:dbl[])
                n3391 = Initialize Array(w5230, 1 ("dimension size")) -> (w5227:dbl[])
                n3392 = Initialize Array(w5203, 1 ("dimension size")) -> (w5208:dbl[])
                n3393 = Initialize Array(w5175, 1 ("dimension size")) -> (w5177:dbl[])
                n3394 = Select(t=w5192, s=w5169, f=w5193) -> (s? t:f=w5190:dbl[])
                "Saved trap pos" <- w5190
                n3395 = feedback-in #41(w5190) -> ()
                n3396 = feedback #42(w5227) -> (w5228:dbl[])
                n3397 = Build Array (concatenate)(w5228, w5227) -> (w5226:dbl[])
                n3398 = feedback #43(w5208) -> (w5209:dbl[])
                n3399 = feedback #44(w5177) -> (w5178:dbl[])
                n3400 = Build Array (concatenate)(w5209, w5208) -> (w5207:dbl[])
                n3401 = Build Array (concatenate)(w5178, w5177) -> (w5176:dbl[])
                n3402 = Select(t=w5227, s=w5169, f=w5226) -> (s? t:f=w5206:dbl[])
                n3403 = feedback-in #42(w5206) -> ()
                n3404 = Select(t=w5208, s=w5169, f=w5207) -> (s? t:f=w5205:dbl[])
                n3405 = feedback-in #43(w5205) -> ()
                n3406 = Select(t=w5177, s=w5169, f=w5176) -> (s? t:f=w5170:dbl[])
                n3407 = feedback-in #44(w5170) -> ()
                n3408 = Build Array(w5206, w5205, w5170) -> (→"Save APD Deriv":dbl[][])
              }
            }
            "Progress" <- w5152
            "Progress 2" <- w5152
          }
        }
      }
    }
    n3409 = local read "wait to reset values"() -> (w3804:bool)
    n3410 = Not(x=w3802) -> (.not. x?=w3805:bool)
    n3411 = And(x=w3805, y=w3804) -> (x .and. y?=w3806:bool)
    n3412 = case "Part of MCL raster scanning: returns to initial positions after scan done" shown="True" w3806 {
      tunnel: w3539 -> [w4680 w4687]
      tunnel: [w4680 w4686] -> w3808
      tunnel: w3538 -> [w4679 w4685]
      tunnel: [w4679 w4684] -> w3803
      frame False {
      }
      frame True {
        w4695 = 10.0 ("y")
        w4694 = 32767.0 ("y")
        # "to return scan values\nafter a synchronous \nAOM scan"
        n3413 = local read "AO2"() -> (w4688:dbl)
        n3414 = local read "AO1"() -> (w4689:dbl)
        n3415 = local write "wait to reset values"(FALSE ("wait to reset values")) -> ()
        n3416 = Multiply(x=w4689, y=w4694) -> (x*y=w4691:dbl)
        n3417 = Multiply(x=w4688, y=w4694) -> (x*y=w4693:dbl)
        n3418 = Divide(x=w4691, y=w4695) -> (x/y=w4690:dbl)
        n3419 = Divide(x=w4693, y=w4695) -> (x/y=w4692:dbl)
        n3420 = To Word Integer(number=w4690) -> (16bit integer=w4696:i16)
        n3421 = To Word Integer(number=w4692) -> (16bit integer=w4697:i16)
        n3422 = local read "Total Counts (ticks)"() -> (w4681:u16)
        n3423 = xnode "Read/Write Control"("FPGA VI Reference In"=w4687, "error in"=w4685, "AO1"=w4696, "AO2"=w4697, "MCL count"=w4681) -> ("FPGA VI Reference Out"=w4686:T20, "error out"=w4684:errorcluster)
        n3424 = local read "Scan Range (V)\n(of steps)"() -> (w4682:dbl)
        n3425 = property on="Scan Range (V)\n(of steps)" class="DigNum (strict)"("Val(Sgnl)"=w4682) -> ()  [unwired: 2 in, 2 out]
      }
    }
    n3426 = node-c288() -> ()  [unwired: 2 out]
  }
  n3427 = node-c288(w21) -> ()  [unwired: 1 out]
  n3428 = node-c288(w65) -> ()  [unwired: 1 out]
  n3429 = node-c288(w67) -> ()  [unwired: 1 out]
  n3430 = property on="Saved trap pos" class="WFGraph (strict)"("Visible"=FALSE) -> ()  [unwired: 2 in, 2 out]
  n3431 = property on="Trap Delta Graph" class="WFGraph (strict)"("Visible"=TRUE) -> ()  [unwired: 2 in, 2 out]
  n3432 = local write "Trap pos"(FALSE ("Trap pos")) -> ()
  n3433 = node-c288(w53) -> ()  [unwired: 1 out]
  n3434 = disable-structure shown="Disabled" {
    disable-tunnel: w57 -> [w5303 _]
    disable-tunnel: w56 -> [w5302 _]
    frame Disabled {
      n3435 = VISA Close(VISA resource name=w5303, error in (no error)=w5302) -> (error out=w5304:errorcluster)
      n3436 = call <vilib>:"Simple Error Handler.vi"("error in (no error)"=w5304) -> ()  [unwired: 1 in, 8 out]
    }
    frame Enabled {
    }
  }
  n3437 = node-c288(w63) -> ()  [unwired: 1 out]
  n3438 = node-c288(w72) -> ()  [unwired: 1 out]
  n3439 = flat-sequence {
    tunnel: w79 -> [w5308]
    tunnel: w80 -> [w5309]
    tunnel: [w5307] -> w78
    tunnel: [w5306] -> w77
    tunnel: w76 -> [_]
    tunnel: w74 -> [_]
    tunnel: w69 -> [_]
    tunnel: w78 -> [w5310]
    tunnel: w77 -> [w5311]
    frame #0 {
      w5305 = FALSE ("AI to FIFO")
      n3440 = xnode "Read/Write Control"("FPGA VI Reference In"=w5309, "error in"=w5308, "AI to FIFO"=w5305, "APD to FIFO"=w5305) -> ("FPGA VI Reference Out"=w5307:T20, "error out"=w5306:errorcluster)
    }
    frame #1 {
      n3441 = xnode "Close FPGA VI Reference"("FPGA VI Reference In"=w5310, "error in"=w5311) -> ("error out"=→"error out":errorcluster)
    }
  }
